vi "Dresden R2R Sputter 03.02.2018 IY24.vi"() -> ()   [LabVIEW 2009] (continued)
                          n12072 = Or(x=w18799, y=w18797) -> (x .or. y?=w18798:bool)
                        }
                      }
                      frame #1 {
                      }
                    }
                  }
                  frame #2 {
                    n12073 = local read "Semi"() -> (w18807:bool)
                    n12074 = case shown="False" w18807 {
                      frame #0 {
                        n12075 = local write "Cassette_servo_speed_value"(u16 100 ("Cassette_servo_speed_value")) -> ()
                      }
                      frame #1 {
                      }
                    }
                  }
                  frame #3 {
                    n12076 = local read "Semi"() -> (w18809:bool)
                    n12077 = case shown="False" w18809 {
                      frame #0 {
                        n12078 = Wait (ms)(milliseconds to wait=u32 200 ("millisecond multiple")) -> ()  [unwired: 1 out]
                      }
                      frame #1 {
                      }
                    }
                  }
                  frame #4 {
                    n12079 = local read "Semi"() -> (w18811:bool)
                    n12080 = case shown="False" w18811 {
                      frame #0 {
                        n12081 = local write "Cassette_servo_speed_auto_set"(TRUE ("Cassette_servo_speed_auto_set")) -> ()
                      }
                      frame #1 {
                      }
                    }
                  }
                  frame #5 {
                    n12082 = local read "Semi"() -> (w18813:bool)
                    n12083 = case shown="False" w18813 {
                      frame #0 {
                        n12084 = Wait (ms)(milliseconds to wait=u32 200 ("millisecond multiple")) -> ()  [unwired: 1 out]
                      }
                      frame #1 {
                      }
                    }
                  }
                  frame #6 {
                    n12085 = while {
                      i -> [w18818]
                      stop <- w18815 stop-if-true
                      n12086 = Greater?(x=w18818, y=50) -> (0:w18819:bool)
                      n12087 = local read "Cnt_Right_slow_di"() -> (w18821:bool)
                      n12088 = case shown="True" w18819 {
                        frame #0 {
                        }
                        frame #1 {
                          n12089 = local write "Semi"(TRUE ("Semi")) -> ()
                          n12090 = local write "Error Message"("\nPlease check connections." ("Error Message")) -> ()
                        }
                      }
                      n12091 = case shown="False" w18821 {
                        tunnel: [FALSE ("Cnt_Left_slow_do") TRUE ("Cnt_Left_slow_do")] -> w18817
                        frame #0 {
                          n12092 = local write "Cnt_Right_slow_do"(TRUE ("Cnt_Left_slow_do")) -> ()
                          n12093 = Wait Until Next ms Multiple(millisecond multiple=u32 200) -> ()  [unwired: 1 out]
                        }
                        frame #1 {
                        }
                      }
                      n12094 = local read "Semi"() -> (w18816:bool)
                      n12095 = Or(x=w18817, y=w18816) -> (x .or. y?=w18815:bool)
                    }
                  }
                  frame #7 {
                    n12096 = local read "Semi"() -> (w18828:bool)
                    n12097 = case shown="False" w18828 {
                      frame #0 {
                        n12098 = local write "CH1_2trns_12"(TRUE ("CH1_2trns_11")) -> ()
                        n12099 = Wait (ms)(milliseconds to wait=u32 500) -> ()  [unwired: 1 out]
                      }
                      frame #1 {
                      }
                    }
                  }
                }
              }
              frame #1 {
              }
            }
          }
          frame #18 {
            # "CASETTE STOP AND FIX"
            n12100 = local read "Semi"() -> (w18831:bool)
            n12101 = case shown="False" w18831 {
              frame #0 {
                n12102 = stacked-sequence {
                  frame #0 {
                    # "Center Casette stop"
                    n12103 = local read "Semi"() -> (w18832:bool)
                    n12104 = case shown="False" w18832 {
                      frame #0 {
                        n12105 = stacked-sequence {
                          frame #0 {
                            n12106 = while {
                              i -> [w18839]
                              stop <- w18834 stop-if-true
                              n12107 = local read "Ch1_Right_limit_di"() -> (w18833:bool)
                              n12108 = Greater?(x=w18839, y=600) -> (0:w18837:bool)
                              n12109 = case shown="True" w18837 {
                                frame #0 {
                                }
                                frame #1 {
                                n12110 = local write "Semi"(TRUE ("Semi")) -> ()
                                n12111 = local write "Error Message"("Transfer process was cancelled.\nPlease check Casette connections." ("Error Message")) -> ()
                                }
                              }
                              n12112 = case shown="False" w18833 {
                                tunnel: [FALSE TRUE] -> w18836
                                frame #0 {
                                n12113 = Wait Until Next ms Multiple(millisecond multiple=u32 200) -> ()  [unwired: 1 out]
                                }
                                frame #1 {
                                }
                              }
                              n12114 = local read "Semi"() -> (w18835:bool)
                              n12115 = Or(x=w18836, y=w18835) -> (x .or. y?=w18834:bool)
                            }
                          }
                          frame #1 {
                            n12116 = disable-structure shown="Disabled" {
                              frame #0 {
                                n12117 = while {
                                i -> [w18854]
                                stop <- w18849 stop-if-true
                                n12118 = local read "Counter_read_data"() -> (w18846:i16)
                                n12119 = Greater?(x=w18854, y=5000) -> (0:w18852:bool)
                                n12120 = case shown="True" w18852 {
                                frame #0 {
                                }
                                frame #1 {
                                n12121 = local write "Semi"(TRUE ("Semi")) -> ()
                                n12122 = local write "Error Message"("Transfer process was cancelled.\nPlease check Casette connections." ("Error Message")) -> ()
                                }
                                }
                                n12123 = In Range and Coerce(upper limit=i16 2209, x=w18846, lower limit=i16 2199 ("upper limit")) -> (In Range?=w18845:bool)  [unwired: 1 out]
                                n12124 = case shown="True" w18845 {
                                tunnel: [FALSE TRUE] -> w18851
                                frame #0 {
                                }
                                frame #1 {
                                n12125 = Wait Until Next ms Multiple(millisecond multiple=u32 500) -> ()  [unwired: 1 out]
                                }
                                }
                                n12126 = local read "Semi"() -> (w18850:bool)
                                n12127 = Or(x=w18851, y=w18850) -> (x .or. y?=w18849:bool)
                                }
                              }
                              frame #1 {
                              }
                            }
                          }
                          frame #2 {
                            n12128 = while {
                              i -> [w18866]
                              stop <- w18861 stop-if-true
                              n12129 = local read "Casette_servo_start/stop_di"() -> (w18860:bool)
                              n12130 = Greater?(x=w18866, y=50) -> (0:w18864:bool)
                              n12131 = case shown="True" w18864 {
                                frame #0 {
                                }
                                frame #1 {
                                n12132 = local write "Semi"(TRUE ("Semi")) -> ()
                                n12133 = local write "Error Message"("Transfer process was cancelled.\nPlease check Casette connections." ("Error Message")) -> ()
                                }
                              }
                              n12134 = case shown="True" w18860 {
                                tunnel: [TRUE FALSE] -> w18863
                                frame #0 {
                                }
                                frame #1 {
                                n12135 = Wait Until Next ms Multiple(millisecond multiple=u32 200) -> ()  [unwired: 1 out]
                                n12136 = local write "Casette_servo_start/stop_do"(FALSE ("Casette_servo_start/stop_di")) -> ()
                                }
                              }
                              n12137 = local read "Semi"() -> (w18862:bool)
                              n12138 = Or(x=w18863, y=w18862) -> (x .or. y?=w18861:bool)
                            }
                          }
                          frame #3 {
                            n12139 = local read "Semi"() -> (w18873:bool)
                            n12140 = case shown="False" w18873 {
                              frame #0 {
                                n12141 = Wait (ms)(milliseconds to wait=u32 200) -> ()  [unwired: 1 out]
                              }
                              frame #1 {
                              }
                            }
                          }
                          frame #4 {
                            n12142 = local read "Semi"() -> (w18875:bool)
                            n12143 = case shown="False" w18875 {
                              frame #0 {
                                n12144 = local write "Cassette_servo_speed_value"(u16 0 ("Cassette_servo_speed_value")) -> ()
                              }
                              frame #1 {
                              }
                            }
                          }
                          frame #5 {
                            n12145 = local read "Semi"() -> (w18877:bool)
                            n12146 = case shown="False" w18877 {
                              frame #0 {
                                n12147 = Wait (ms)(milliseconds to wait=u32 200) -> ()  [unwired: 1 out]
                              }
                              frame #1 {
                              }
                            }
                          }
                          frame #6 {
                            n12148 = local read "Semi"() -> (w18879:bool)
                            n12149 = case shown="False" w18879 {
                              frame #0 {
                                n12150 = local write "Cassette_servo_speed_auto_set"(TRUE ("Cassette_servo_speed_auto_set")) -> ()
                              }
                              frame #1 {
                              }
                            }
                          }
                          frame #7 {
                            n12151 = local read "Semi"() -> (w18881:bool)
                            n12152 = case shown="False" w18881 {
                              frame #0 {
                                n12153 = Wait (ms)(milliseconds to wait=u32 200) -> ()  [unwired: 1 out]
                              }
                              frame #1 {
                              }
                            }
                          }
                          frame #8 {
                            n12154 = local read "Semi"() -> (w18883:bool)
                            n12155 = case shown="False" w18883 {
                              frame #0 {
                                n12156 = local write "CH1_2trns_13"(TRUE ("CH1_2trns_9")) -> ()
                                n12157 = Wait (ms)(milliseconds to wait=u32 500) -> ()  [unwired: 1 out]
                              }
                              frame #1 {
                              }
                            }
                          }
                        }
                      }
                      frame #1 {
                      }
                    }
                  }
                  frame #1 {
                    # "CASETTE FIX DOWN CH2"
                    n12158 = local read "Semi"() -> (w18886:bool)
                    n12159 = case shown="False" w18886 {
                      frame #0 {
                        n12160 = stacked-sequence {
                          frame #0 {
                            n12161 = local read "Semi"() -> (w18887:bool)
                            n12162 = case shown="False" w18887 {
                              frame #0 {
                                n12163 = while {
                                i -> [w18894]
                                stop <- w18889 stop-if-true
                                n12164 = Greater?(x=w18894, y=50) -> (0:w18892:bool)
                                n12165 = local read "Ch1_Cst_fix_down_di"() -> (w18888:bool)
                                n12166 = case shown="True" w18892 {
                                frame #0 {
                                }
                                frame #1 {
                                n12167 = local write "Semi"(TRUE ("Semi")) -> ()
                                n12168 = local write "Error Message"("Up/Down positions could not reach\nthe down position.\nPlease check connections." ("Error Message")) -> ()
                                }
                                }
                                n12169 = case shown="False" w18888 {
                                tunnel: [FALSE TRUE] -> w18891
                                frame #0 {
                                n12170 = Wait Until Next ms Multiple(millisecond multiple=u32 200) -> ()  [unwired: 1 out]
                                n12171 = local write "Ch1_Cst_fix_do"(TRUE ("Ch1_pet_cool_up_do")) -> ()
                                }
                                frame #1 {
                                }
                                }
                                n12172 = local read "Semi"() -> (w18890:bool)
                                n12173 = Or(x=w18891, y=w18890) -> (x .or. y?=w18889:bool)
                                }
                              }
                              frame #1 {
                              }
                            }
                          }
                          frame #1 {
                            n12174 = local read "Semi"() -> (w18901:bool)
                            n12175 = case shown="False" w18901 {
                              frame #0 {
                                n12176 = local write "CH1_2trns_14"(TRUE ("CH1_2trns_9")) -> ()
                                n12177 = Wait (ms)(milliseconds to wait=u32 500) -> ()  [unwired: 1 out]
                              }
                              frame #1 {
                              }
                            }
                          }
                        }
                      }
                      frame #1 {
                      }
                    }
                  }
                  frame #2 {
                    n12178 = local read "Semi"() -> (w18904:bool)
                    n12179 = case shown="False" w18904 {
                      frame #0 {
                        n12180 = stacked-sequence {
                          frame #0 {
                            n12181 = local read "Semi"() -> (w18905:bool)
                            n12182 = case shown="False" w18905 {
                              frame #0 {
                                n12183 = while {
                                i -> [w18912]
                                stop <- w18907 stop-if-true
                                n12184 = Greater?(x=w18912, y=50) -> (0:w18910:bool)
                                n12185 = local read "Ch1_Trns_gv_bp2_di"() -> (w18906:bool)
                                n12186 = case shown="True" w18910 {
                                frame #0 {
                                }
                                frame #1 {
                                n12187 = local write "Semi"(TRUE ("Semi")) -> ()
                                n12188 = local write "Error Message"("Transfer process was cancelled.\nPlease check CH1-Trns-GV connections." ("Error Message")) -> ()
                                }
                                }
                                n12189 = case shown="True" w18906 {
                                tunnel: [TRUE FALSE] -> w18909
                                frame #0 {
                                }
                                frame #1 {
                                n12190 = Wait Until Next ms Multiple(millisecond multiple=u32 200) -> ()  [unwired: 1 out]
                                n12191 = local write "Ch1_Trns_gv_bp2_do"(FALSE ("Ch1_pet_cool_up_do")) -> ()
                                }
                                }
                                n12192 = local read "Semi"() -> (w18908:bool)
                                n12193 = Or(x=w18909, y=w18908) -> (x .or. y?=w18907:bool)
                                }
                              }
                              frame #1 {
                              }
                            }
                          }
                          frame #1 {
                            n12194 = local read "Semi"() -> (w18919:bool)
                            n12195 = case shown="False" w18919 {
                              frame #0 {
                                n12196 = Wait (ms)(milliseconds to wait=u32 500) -> ()  [unwired: 1 out]
                              }
                              frame #1 {
                              }
                            }
                          }
                          frame #2 {
                            n12197 = local read "Semi"() -> (w18921:bool)
                            n12198 = case shown="False" w18921 {
                              frame #0 {
                                n12199 = while {
                                i -> [w18928]
                                stop <- w18923 stop-if-true
                                n12200 = Greater?(x=w18928, y=50) -> (0:w18926:bool)
                                n12201 = local read "Ch2_trns_gv_bp_di"() -> (w18922:bool)
                                n12202 = case shown="True" w18926 {
                                frame #0 {
                                }
                                frame #1 {
                                n12203 = local write "Semi"(TRUE ("Semi")) -> ()
                                n12204 = local write "Error Message"("Transfer process was cancelled.\nPlease check CH1-Trns-GV connections." ("Error Message")) -> ()
                                }
                                }
                                n12205 = case shown="True" w18922 {
                                tunnel: [TRUE FALSE] -> w18925
                                frame #0 {
                                }
                                frame #1 {
                                n12206 = Wait Until Next ms Multiple(millisecond multiple=u32 200) -> ()  [unwired: 1 out]
                                n12207 = local write "Ch2_trns_gv_bp_do"(FALSE ("Ch1_pet_cool_up_do")) -> ()
                                }
                                }
                                n12208 = local read "Semi"() -> (w18924:bool)
                                n12209 = Or(x=w18925, y=w18924) -> (x .or. y?=w18923:bool)
                                }
                              }
                              frame #1 {
                              }
                            }
                          }
                          frame #3 {
                            n12210 = local read "Semi"() -> (w18935:bool)
                            n12211 = case shown="False" w18935 {
                              frame #0 {
                                n12212 = Wait (ms)(milliseconds to wait=u32 500) -> ()  [unwired: 1 out]
                              }
                              frame #1 {
                              }
                            }
                          }
                        }
                      }
                      frame #1 {
                      }
                    }
                  }
                  frame #3 {
                    n12213 = local read "Semi"() -> (w18937:bool)
                    n12214 = case shown="False" w18937 {
                      frame #0 {
                        n12215 = stacked-sequence {
                          frame #0 {
                            n12216 = local read "Semi"() -> (w18938:bool)
                            n12217 = case shown="False" w18938 {
                              frame #0 {
                                n12218 = local write "Ch1_Trns_gv_open_do"(FALSE ("Ch1_pet_cool_up_do")) -> ()
                              }
                              frame #1 {
                              }
                            }
                          }
                          frame #1 {
                            n12219 = local read "Semi"() -> (w18940:bool)
                            n12220 = case shown="False" w18940 {
                              frame #0 {
                                n12221 = while {
                                i -> [w18947]
                                stop <- w18942 stop-if-true
                                n12222 = Greater?(x=w18947, y=500) -> (0:w18945:bool)
                                n12223 = local read "Ch1_Trns_gv_close_di"() -> (w18941:bool)
                                n12224 = case shown="True" w18945 {
                                frame #0 {
                                }
                                frame #1 {
                                n12225 = local write "Semi"(TRUE ("Semi")) -> ()
                                n12226 = local write "Error Message"("Transfer process was cancelled.\nPlease check  GV connections." ("Error Message")) -> ()
                                }
                                }
                                n12227 = case shown="False" w18941 {
                                tunnel: [FALSE TRUE] -> w18944
                                frame #0 {
                                n12228 = Wait Until Next ms Multiple(millisecond multiple=u32 200) -> ()  [unwired: 1 out]
                                n12229 = local write "Ch1_Trns_gv_close_do"(TRUE ("Ch1_pet_cool_up_do")) -> ()
                                }
                                frame #1 {
                                }
                                }
                                n12230 = local read "Semi"() -> (w18943:bool)
                                n12231 = Or(x=w18944, y=w18943) -> (x .or. y?=w18942:bool)
                                }
                              }
                              frame #1 {
                              }
                            }
                          }
                          frame #2 {
                            n12232 = local read "Semi"() -> (w18954:bool)
                            n12233 = case shown="False" w18954 {
                              frame #0 {
                                n12234 = local write "CH1_2trns_17"(TRUE ("CH1_2trns_9")) -> ()
                                n12235 = Wait (ms)(milliseconds to wait=u32 500) -> ()  [unwired: 1 out]
                              }
                              frame #1 {
                              }
                            }
                          }
                        }
                      }
                      frame #1 {
                      }
                    }
                  }
                  frame #4 {
                    # "PET COOL DOWN OF CH2"
                    n12236 = local read "Semi"() -> (w18957:bool)
                    n12237 = case shown="False" w18957 {
                      frame #0 {
                        n12238 = stacked-sequence {
                          frame #0 {
                            n12239 = local read "Semi"() -> (w18958:bool)
                            n12240 = case shown="False" w18958 {
                              frame #0 {
                                n12241 = local write "Ch1_Pet_cool_up_do"(FALSE ("Ch1_pet_cool_up_do")) -> ()
                              }
                              frame #1 {
                              }
                            }
                          }
                          frame #1 {
                            n12242 = local read "Semi"() -> (w18960:bool)
                            n12243 = case shown="False" w18960 {
                              frame #0 {
                                n12244 = while {
                                i -> [w18967]
                                stop <- w18962 stop-if-true
                                n12245 = Greater?(x=w18967, y=300) -> (0:w18965:bool)
                                n12246 = case shown="True" w18965 {
                                frame #0 {
                                }
                                frame #1 {
                                n12247 = local write "Semi"(TRUE ("Semi")) -> ()
                                n12248 = local write "Error Message"("SBS Cool Up/Down positions could not reach\nthe down position.\nPlease check connections." ("Error Message")) -> ()
                                }
                                }
                                n12249 = local read "Ch1_Pet_cool_down_di"() -> (w18961:bool)
                                n12250 = case shown="False" w18961 {
                                tunnel: [FALSE TRUE] -> w18964
                                frame #0 {
                                n12251 = Wait Until Next ms Multiple(millisecond multiple=u32 200) -> ()  [unwired: 1 out]
                                n12252 = local write "Ch1_Pet_cool_down_do"(TRUE ("Ch1_pet_cool_up_do")) -> ()
                                }
                                frame #1 {
                                }
                                }
                                n12253 = local read "Semi"() -> (w18963:bool)
                                n12254 = Or(x=w18964, y=w18963) -> (x .or. y?=w18962:bool)
                                }
                              }
                              frame #1 {
                              }
                            }
                          }
                          frame #2 {
                            n12255 = local read "Semi"() -> (w18974:bool)
                            n12256 = case shown="False" w18974 {
                              frame #0 {
                                n12257 = local write "CH1_2trns_15"(TRUE ("CH1_2trns_9")) -> ()
                                n12258 = Wait (ms)(milliseconds to wait=u32 500) -> ()  [unwired: 1 out]
                              }
                              frame #1 {
                              }
                            }
                          }
                        }
                      }
                      frame #1 {
                      }
                    }
                  }
                  frame #5 {
                    # "SRV PIS FOR"
                    n12259 = local read "Semi"() -> (w18977:bool)
                    n12260 = case shown="False" w18977 {
                      frame #0 {
                        n12261 = stacked-sequence {
                          frame #0 {
                            n12262 = local read "Semi"() -> (w18978:bool)
                            n12263 = case shown="False" w18978 {
                              frame #0 {
                                n12264 = local write "Ch1_SRV1_PIST_Back_do"(FALSE ("Ch1_pet_cool_up_do")) -> ()
                              }
                              frame #1 {
                              }
                            }
                          }
                          frame #1 {
                            n12265 = local read "Semi"() -> (w18980:bool)
                            n12266 = case shown="False" w18980 {
                              frame #0 {
                                n12267 = while {
                                i -> [w18987]
                                stop <- w18982 stop-if-true
                                n12268 = Greater?(x=w18987, y=100) -> (0:w18985:bool)
                                n12269 = local read "Ch1_SRV1_PIST For_di"() -> (w18981:bool)
                                n12270 = case shown="True" w18985 {
                                frame #0 {
                                }
                                frame #1 {
                                n12271 = local write "Semi"(TRUE ("Semi")) -> ()
                                n12272 = local write "Error Message"("For/Back positions could not reach\nthe forward position.\nPlease check connections." ("Error Message")) -> ()
                                }
                                }
                                n12273 = case shown="False" w18981 {
                                tunnel: [FALSE TRUE] -> w18984
                                frame #0 {
                                n12274 = Wait Until Next ms Multiple(millisecond multiple=u32 200) -> ()  [unwired: 1 out]
                                n12275 = local write "Ch1_SRV1_PIST For_do"(TRUE ("Ch1_pet_cool_up_do")) -> ()
                                }
                                frame #1 {
                                }
                                }
                                n12276 = local read "Semi"() -> (w18983:bool)
                                n12277 = Or(x=w18984, y=w18983) -> (x .or. y?=w18982:bool)
                                }
                              }
                              frame #1 {
                              }
                            }
                          }
                          frame #2 {
                            n12278 = local read "Semi"() -> (w18994:bool)
                            n12279 = case shown="False" w18994 {
                              frame #0 {
                                n12280 = local write "CH1_2trns_16"(TRUE ("CH1_2trns_9")) -> ()
                                n12281 = Wait (ms)(milliseconds to wait=u32 500) -> ()  [unwired: 1 out]
                              }
                              frame #1 {
                              }
                            }
                          }
                        }
                      }
                      frame #1 {
                      }
                    }
                  }
                }
              }
              frame #1 {
              }
            }
          }
          frame #19 {
            # "Sensors deactive"
            n12282 = local read "Semi"() -> (w18997:bool)
            n12283 = case shown="False" w18997 {
              frame #0 {
                n12284 = stacked-sequence {
                  frame #0 {
                    n12285 = local read "Semi"() -> (w18998:bool)
                    n12286 = case shown="False" w18998 {
                      frame #0 {
                        n12287 = while {
                          i -> [w19001]
                          stop <- w19002 stop-if-true
                          n12288 = Greater?(x=w19001, y=50) -> (0:w18999:bool)
                          n12289 = local read "Cnt_Right_slow_di"() -> (w19005:bool)
                          n12290 = case shown="True" w18999 {
                            frame #0 {
                            }
                            frame #1 {
                              n12291 = local write "Semi"(TRUE ("Semi")) -> ()
                              n12292 = local write "Error Message"("Transfer process was\ncancelled.Please check right slow sensor." ("Error Message")) -> ()
                            }
                          }
                          n12293 = case shown="False" w19005 {
                            tunnel: [FALSE ("Ch1_pet_cool_up_do") TRUE ("Ch1_pet_cool_up_do")] -> w19004
                            frame #0 {
                              n12294 = Wait Until Next ms Multiple(millisecond multiple=u32 200) -> ()  [unwired: 1 out]
                              n12295 = local write "Cnt_Right_slow_do"(TRUE ("Ch1_pet_cool_up_do")) -> ()
                            }
                            frame #1 {
                            }
                          }
                          n12296 = local read "Semi"() -> (w19003:bool)
                          n12297 = Or(x=w19004, y=w19003) -> (x .or. y?=w19002:bool)
                        }
                      }
                      frame #1 {
                      }
                    }
                  }
                  frame #1 {
                    n12298 = local read "Semi"() -> (w19012:bool)
                    n12299 = case shown="False" w19012 {
                      frame #0 {
                        n12300 = while {
                          i -> [w19015]
                          stop <- w19016 stop-if-true
                          n12301 = Greater?(x=w19015, y=50) -> (0:w19013:bool)
                          n12302 = local read "Cnt_Right_limit_di"() -> (w19019:bool)
                          n12303 = case shown="True" w19013 {
                            frame #0 {
                            }
                            frame #1 {
                              n12304 = local write "Semi"(TRUE ("Semi")) -> ()
                              n12305 = local write "Error Message"("Transfer process was\ncancelled.Please check right limit sensor." ("Error Message")) -> ()
                            }
                          }
                          n12306 = case shown="False" w19019 {
                            tunnel: [FALSE ("Ch1_pet_cool_up_do") TRUE ("Ch1_pet_cool_up_do")] -> w19018
                            frame #0 {
                              n12307 = Wait Until Next ms Multiple(millisecond multiple=u32 200) -> ()  [unwired: 1 out]
                              n12308 = local write "Cnt_Right_limit_do"(TRUE ("Ch1_pet_cool_up_do")) -> ()
                            }
                            frame #1 {
                            }
                          }
                          n12309 = local read "Semi"() -> (w19017:bool)
                          n12310 = Or(x=w19018, y=w19017) -> (x .or. y?=w19016:bool)
                        }
                      }
                      frame #1 {
                      }
                    }
                  }
                  frame #2 {
                    n12311 = local read "Semi"() -> (w19026:bool)
                    n12312 = case shown="False" w19026 {
                      frame #0 {
                        n12313 = while {
                          i -> [w19029]
                          stop <- w19030 stop-if-true
                          n12314 = Greater?(x=w19029, y=50) -> (0:w19027:bool)
                          n12315 = local read "Cnt_Left_slow_di"() -> (w19033:bool)
                          n12316 = case shown="True" w19027 {
                            frame #0 {
                            }
                            frame #1 {
                              n12317 = local write "Semi"(TRUE ("Semi")) -> ()
                              n12318 = local write "Error Message"("Transfer process was\ncancelled.Please check left slow sensor." ("Error Message")) -> ()
                            }
                          }
                          n12319 = case shown="False" w19033 {
                            tunnel: [FALSE ("Ch1_pet_cool_up_do") TRUE ("Ch1_pet_cool_up_do")] -> w19032
                            frame #0 {
                              n12320 = Wait Until Next ms Multiple(millisecond multiple=u32 200) -> ()  [unwired: 1 out]
                              n12321 = local write "Cnt_Left_slow_do"(TRUE ("Ch1_pet_cool_up_do")) -> ()
                            }
                            frame #1 {
                            }
                          }
                          n12322 = local read "Semi"() -> (w19031:bool)
                          n12323 = Or(x=w19032, y=w19031) -> (x .or. y?=w19030:bool)
                        }
                      }
                      frame #1 {
                      }
                    }
                  }
                  frame #3 {
                    n12324 = local read "Semi"() -> (w19040:bool)
                    n12325 = case shown="False" w19040 {
                      frame #0 {
                        n12326 = while {
                          i -> [w19043]
                          stop <- w19044 stop-if-true
                          n12327 = Greater?(x=w19043, y=50) -> (0:w19041:bool)
                          n12328 = local read "Cnt_Left_limit_di"() -> (w19047:bool)
                          n12329 = case shown="True" w19041 {
                            frame #0 {
                            }
                            frame #1 {
                              n12330 = local write "Semi"(TRUE ("Semi")) -> ()
                              n12331 = local write "Error Message"("Transfer process was\ncancelled.Please check left limit sensor." ("Error Message")) -> ()
                            }
                          }
                          n12332 = case shown="False" w19047 {
                            tunnel: [FALSE ("Ch1_pet_cool_up_do") TRUE ("Ch1_pet_cool_up_do")] -> w19046
                            frame #0 {
                              n12333 = Wait Until Next ms Multiple(millisecond multiple=u32 200) -> ()  [unwired: 1 out]
                              n12334 = local write "Cnt_Left_limit_do"(TRUE ("Ch1_pet_cool_up_do")) -> ()
                            }
                            frame #1 {
                            }
                          }
                          n12335 = local read "Semi"() -> (w19045:bool)
                          n12336 = Or(x=w19046, y=w19045) -> (x .or. y?=w19044:bool)
                        }
                      }
                      frame #1 {
                      }
                    }
                  }
                  frame #4 {
                    n12337 = local read "Semi"() -> (w19054:bool)
                    n12338 = case shown="False" w19054 {
                      frame #0 {
                        n12339 = local write "CH1_2trns_18"(TRUE ("CH1_2trns_7")) -> ()
                        n12340 = Wait (ms)(milliseconds to wait=u32 500) -> ()  [unwired: 1 out]
                      }
                      frame #1 {
                      }
                    }
                  }
                }
              }
              frame #1 {
              }
            }
          }
          frame #20 {
            n12341 = local read "Semi"() -> (w19057:bool)
            n12342 = case shown="False" w19057 {
              frame #0 {
                n12343 = local write "CH1_2trns_19"(TRUE ("CH1_2trns_18")) -> ()
                n12344 = local write "Cnt_Do_Buzzer"(TRUE ("Transfer_ch1_2")) -> ()
                n12345 = Wait (ms)(milliseconds to wait=u32 1500) -> ()  [unwired: 1 out]
              }
              frame #1 {
              }
            }
          }
          frame #21 {
            n12346 = local read "Semi"() -> (w19061:bool)
            n12347 = case shown="False" w19061 {
              frame #0 {
                n12348 = local write "ch_present_position"(1.0 ("ch_present_position")) -> ()
                n12349 = local write "Transfer_ch2_1"(FALSE ("Transfer_ch1_2")) -> ()
                n12350 = local write "Cnt_Do_Buzzer"(FALSE ("Transfer_ch1_2")) -> ()
                n12351 = Wait (ms)(milliseconds to wait=u32 500) -> ()  [unwired: 1 out]
              }
              frame #1 {
              }
            }
          }
        }
      }
      frame #3 {
        n12352 = stacked-sequence {
          frame #0 {
            n12353 = Wait (ms)(milliseconds to wait=u32 1500) -> ()  [unwired: 1 out]
            n12354 = local write "Clean_trnsfr_2_3"(TRUE ("Clean_trnsfr_1_2")) -> ()
            n12355 = local write "system_status"("Chamber 2 to Chamber 3 Transfer Process in Progress." ("system_status")) -> ()
            n12356 = local write "final_process_messages"("Chamber 2 to Chamber 3  Transfer Process was completed." ("final_process_messages")) -> ()
          }
          frame #1 {
            n12357 = stacked-sequence {
              frame #0 {
                n12358 = local write "Routine_check_transfer"(TRUE ("Routine_check_transfer")) -> ()
                n12359 = Wait (ms)(milliseconds to wait=u32 100) -> ()  [unwired: 1 out]
              }
              frame #1 {
                n12360 = while {
                  i -> [w19079]
                  stop <- w19075 stop-if-true
                  n12361 = Greater Or Equal?(x=w19079, y=1500) -> (x >= y?=w19076:bool)
                  n12362 = Wait Until Next ms Multiple(millisecond multiple=u32 200) -> ()  [unwired: 1 out]
                  n12363 = case shown="True" w19076 {
                    frame #0 {
                    }
                    frame #1 {
                      # "Hata mesajı"
                      n12364 = local write "Semi"(TRUE ("Semi")) -> ()
                    }
                  }
                  n12365 = local read "Routine_check_transfer"() -> (w19072:bool)
                  n12366 = local read "Semi"() -> (w19074:bool)
                  n12367 = Not(x=w19072) -> (.not. x?=w19073:bool)
                  n12368 = Or(x=w19073, y=w19074) -> (x .or. y?=w19075:bool)
                }
              }
              frame #2 {
                n12369 = Wait (ms)(milliseconds to wait=u32 500) -> ()  [unwired: 1 out]
              }
            }
          }
          frame #2 {
            # "STARTED UP CH3"
            n12370 = disable-structure shown="Disabled" {
              frame #0 {
                n12371 = local read "Semi"() -> (w19082:bool)
                n12372 = case shown="False" w19082 {
                  frame #0 {
                    n12373 = local read "started_up_ch3"() -> (w19083:bool)
                    n12374 = case shown="False" w19083 {
                      frame #0 {
                        n12375 = stacked-sequence {
                          frame #0 {
                            n12376 = local read "Semi"() -> (w19084:bool)
                            n12377 = case shown="False" w19084 {
                              frame #0 {
                                n12378 = local write "Start_up_ch3"(TRUE ("Start_up_ch2")) -> ()
                              }
                              frame #1 {
                              }
                            }
                          }
                          frame #1 {
                            n12379 = local read "Semi"() -> (w19086:bool)
                            n12380 = case shown="False" w19086 {
                              frame #0 {
                                n12381 = Wait (ms)(milliseconds to wait=u32 16000) -> ()  [unwired: 1 out]
                              }
                              frame #1 {
                              }
                            }
                          }
                          frame #2 {
                            n12382 = local read "Semi"() -> (w19088:bool)
                            n12383 = case shown="False" w19088 {
                              frame #0 {
                                n12384 = while {
                                i -> [w19093]
                                stop <- w19090 stop-if-true
                                n12385 = Greater?(x=w19093, y=80) -> (0:w19091:bool)
                                n12386 = local read "started_up_ch3"() -> (w19089:bool)
                                n12387 = case shown="True" w19091 {
                                frame #0 {
                                }
                                frame #1 {
                                n12388 = local write "Semi"(TRUE ("Semi")) -> ()
                                n12389 = local write "Error Message"("Chamber 1 Pressure is not suitable  \nfor transfer process!\nPlease check connections." ("Error Message")) -> ()